vi "UHR-Fleezers Control (host) - 12.2.vi"() -> ()   [LabVIEW 2014] (continued)
            n2614 = xnode "Read/Write Control"("FPGA VI Reference In"=w4956, "error in"=w4955, "AI to FIFO"=w4959, "APD to FIFO"=w4959, "Start scan"=w4959, "Start scan (MCL)"=w4959) -> ("FPGA VI Reference Out"=w4961:T22, "error out"=w4960:errorcluster)
          }
        }
        "Raster Scanning..." <- TRUE ("Scanning...")
      }
    }
    n2615 = local read "Flushing P3"() -> (w3736:bool)
    n2616 = case "Keep track of when Harvard Pump 3 is done flushing" shown="True" w3736 {
      frame False {
      }
      frame True {
        n2617 = local read "Flush rate (uL/m) P3"() -> (w4119:dbl)
        n2618 = local read "DMA Update Period (s)"() -> (w4113:dbl)
        n2619 = local read "HP3 Flush Time (s)"() -> (w4127:dbl)
        n2620 = Divide(x=w4119, y=60.0) -> (x/y=w4114:dbl)
        n2621 = feedback #6(0) -> (w4125:i32)
        n2622 = Increment(x=w4125) -> (x+1=w4120:i32)
        n2623 = Divide(x=w4127, y=w4113) -> (x/y=w4121:dbl)
        n2624 = Multiply(x=w4113, y=w4114) -> (x*y=w4112:dbl)
        n2625 = Greater?(x=w4120, y=w4121) -> (0:w4124:bool)
        n2626 = feedback #7(0.0) -> (w4115:dbl)
        n2627 = Compound Arithmetic op=MULTIPLY(w4113, w4120, w4114) -> (→"P3 Flush Volume (uL)":dbl)
        n2628 = case shown="True" w4124 {
          tunnel: w4120 -> [w4128 _]
          tunnel: [w4128 0] -> w4123
          frame False {
          }
          frame True {
            w4129 = FALSE ("Flushing P3")
            n2629 = local write "Inject Pump 3"(w4129) -> ()
            n2630 = local write "Flushing P3"(w4129) -> ()
            n2631 = property on="Clear Volume P3" class="Bool (strict)"("Val(Sgnl)"=TRUE ("Value (Signaling)")) -> ()  [unwired: 2 in, 2 out]
          }
        }
        n2632 = feedback-in #6(w4123) -> ()
        n2633 = Divide(x=w4120, y=w4121) -> (x/y=→"P3 Flushing Bar":dbl)
        n2634 = Add(x=w4112, y=w4115) -> (x+y=w4116:dbl)
        "Total Volume\nFlowed P3 (uL)" <- w4116
        n2635 = feedback-in #7(w4116) -> ()
      }
    }
    n2636 = And(x="Save scans", y=w3954) -> (x .and. y?=w3993:bool)
    n2637 = local read "Flushing samp"() -> (w3729:bool)
    n2638 = case shown="True" w3729 {
      frame False {
      }
      frame True {
        n2639 = local read "DMA Update Period (s)"() -> (w4072:dbl)
        n2640 = local read "Flush rate (mL/m)"() -> (w4084:dbl)
        n2641 = local read "Samp Flush Time (s)"() -> (w4085:dbl)
        n2642 = Divide(x=w4084, y=60.0) -> (x/y=w4071:dbl)
        n2643 = feedback #8(0) -> (w4077:i32)
        n2644 = Increment(x=w4077) -> (x+1=w4076:i32)
        n2645 = Divide(x=w4085, y=w4072) -> (x/y=w4081:dbl)
        n2646 = Multiply(x=w4072, y=w4071) -> (x*y=w4070:dbl)
        n2647 = Greater?(x=w4076, y=w4081) -> (0:w4080:bool)
        n2648 = feedback #9(0.0) -> (w4073:dbl)
        n2649 = Compound Arithmetic op=MULTIPLY(w4072, w4076, w4071) -> (→"Samp Volume (uL)":dbl)
        n2650 = Divide(x=w4076, y=w4081) -> (x/y=→"Samp flush bar":dbl)
        n2651 = case shown="True" w4080 {
          tunnel: [w4086 0] -> w4079
          tunnel: w4076 -> [w4086 _]
          frame False {
          }
          frame True {
            w4089 = FALSE ("Flushing samp")
            n2652 = local write "Sample Channel\nFlow"(w4089) -> ()
            n2653 = local write "Flushing samp"(w4089) -> ()
            n2654 = property on="Clear Volume" class="Bool (strict)"("Val(Sgnl)"=TRUE) -> ()  [unwired: 2 in, 2 out]
          }
        }
        n2655 = feedback-in #8(w4079) -> ()
        n2656 = Add(x=w4070, y=w4073) -> (x+y=w4074:dbl)
        "Total Volume\nFlowed Samp (uL)" <- w4074
        n2657 = feedback-in #9(w4074) -> ()
      }
    }
    n2658 = Compound Arithmetic op=OR("Start MCL Scan", "Confocal\nImage", "Confocal\nLinescan") -> (w3952:bool)
    n2659 = And(x="Save Data (MCL)", y=w3952) -> (x .and. y?=w3992:bool)
    n2660 = case "Start MCL raster scan" shown="True" w3952 {
      tunnel: w3720 -> [w4534 w4550]
      tunnel: w3994 -> [w4533 w4549]
      tunnel: [w4534 w4545] -> w3727
      tunnel: [w4533 w4544] -> w3725
      tunnel: [FALSE w4543] -> w3978
      tunnel: "Start MCL Scan" -> [_ w4538]
      tunnel: "Confocal\nImage" -> [_ w4537]
      tunnel: "Confocal\nLinescan" -> [_ _]
      frame False {
      }
      frame True {
        w4543 = TRUE
        n2661 = case shown="True" "Restart DMA? (MCL)" {
          tunnel: [w4595 w4597] -> w4548
          tunnel: [w4594 w4596] -> w4547
          tunnel: w4550 -> [w4595 w4600]
          tunnel: w4549 -> [w4594 w4599]
          frame False {
          }
          frame True {
            n2662 = call "reset FPGA DMA.vi"("error in"=w4599, "FPGA VI Reference In"=w4600) -> ("error out"=w4596:errorcluster, "FPGA VI Reference Out"=w4597:T22)
            n2663 = local write "Overflow (data lost)"(FALSE ("Overflow (data lost)")) -> ()
          }
        }
        n2664 = case shown="False" w4538 {
          selector: w4538 -> [_ w4554]
          tunnel: w4537 -> [w4553 _]
          tunnel: [w4553 w4554] -> w4536
          frame False {
            n2665 = property on="2D or 1D Scan" class="Bool (strict)"("Val(Sgnl)"=w4553) -> ()  [unwired: 2 in, 2 out]
            n2666 = property on="Confocal\nImage" class="Bool (strict)"("Value"=FALSE ("Start Confocal Map")) -> ()  [unwired: 2 in, 2 out]
          }
          frame True {
          }
        }
        n2667 = local write "MCL Scanning"(w4543) -> ()
        n2668 = local read "AO1"() -> (w4540:dbl)
        n2669 = local read "AO2"() -> (w4539:dbl)
        n2670 = case shown="True" "Center Scan" {
          tunnel: w4548 -> [w4561 w4593]
          tunnel: w4547 -> [w4560 w4592]
          tunnel: [w4559 w4591] -> w4545
          tunnel: [w4558 w4590] -> w4544
          tunnel: [w4556 w4577] -> w4542
          tunnel: [w4555 w4576] -> w4541
          tunnel: w4540 -> [w4556 w4582]
          tunnel: w4539 -> [w4555 w4585]
          tunnel: w4536 -> [_ _]
          frame False {
            w4557 = TRUE ("AI to FIFO")
            n2671 = xnode "Read/Write Control"("FPGA VI Reference In"=w4561, "error in"=w4560, "AI to FIFO"=w4557, "APD to FIFO"=w4557, "Start scan (MCL)"=w4557) -> ("FPGA VI Reference Out"=w4559:T22, "error out"=w4558:errorcluster)
          }
          frame True {
            w4589 = TRUE ("AI to FIFO")
            n2672 = local read "Scan steps (MCL)"() -> (w4568:u64)
            n2673 = local read "Scan lines (y)"() -> (w4564:u64)
            n2674 = local read "Fast Scan Dir"() -> (w4575:bool)
            n2675 = local read "Actual MCL Inc (V)"() -> (w4565:dbl)
            n2676 = Decrement(x=w4564) -> (x-1=w4563:u64)
            n2677 = Decrement(x=w4568) -> (x-1=w4567:u64)
            n2678 = Multiply(x=w4565, y=w4563) -> (x*y=w4562:dbl)
            n2679 = Divide(x=w4562, y=2.0) -> (x/y=w4572:dbl)
            n2680 = Multiply(x=w4565, y=w4567) -> (x*y=w4566:dbl)
            n2681 = Divide(x=w4566, y=2.0) -> (x/y=w4571:dbl)
            n2682 = Select(t=w4571, s=w4575, f=w4572) -> (s? t:f=w4570:dbl)
            n2683 = Select(t=w4572, s=w4575, f=w4571) -> (s? t:f=w4574:dbl)
            n2684 = Subtract(x=w4582, y=w4574) -> (x-y=w4573:dbl)
            n2685 = Subtract(x=w4585, y=w4570) -> (x-y=w4569:dbl)
            n2686 = local read "2D or 1D Scan"() -> (w4587:bool)
            n2687 = Not(x=w4575) -> (.not. x?=w4581:bool)
            n2688 = Not(x=w4587) -> (.not. x?=w4583:bool)
            n2689 = And(x=w4575, y=w4583) -> (x .and. y?=w4584:bool)
            n2690 = And(x=w4583, y=w4581) -> (x .and. y?=w4586:bool)
            n2691 = Select(t=w4585, s=w4586, f=w4569) -> (s? t:f=w4576:dbl)
            n2692 = Select(t=w4582, s=w4584, f=w4573) -> (s? t:f=w4577:dbl)
            n2693 = call "Volt to I16.vi"("Voltage In"=w4577) -> ("I16 Voltage Out"=w4580:i16)
            n2694 = call "Volt to I16.vi"("Voltage In"=w4576) -> ("I16 Voltage Out"=w4579:i16)
            n2695 = xnode "Read/Write Control"("FPGA VI Reference In"=w4593, "error in"=w4592, "AI to FIFO"=w4589, "APD to FIFO"=w4589, "Start scan (MCL)"=w4589, "AO1"=w4580, "AO2"=w4579) -> ("FPGA VI Reference Out"=w4591:T22, "error out"=w4590:errorcluster)
          }
        }
        "Initial Y" <- w4542
        "Initial X" <- w4541
        n2696 = local write "Tab Control 6"(T3."Imaging" ("Tab Control 6")) -> ()
        "wait to reset values" <- w4543
      }
    }
    n2697 = case shown="True" "Wiggle" {
      selector: "Wiggle" -> [w4043 _]
      tunnel: w3727 -> [w4045 w4058]
      tunnel: [w4042 w4061] -> w3726
      tunnel: w3725 -> [w4044 w4056]
      tunnel: [w4041 w4060] -> w3724
      frame False {
        n2698 = xnode "Read/Write Control"("FPGA VI Reference In"=w4045, "error in"=w4044, "Wiggle trap 1"=w4043) -> ("FPGA VI Reference Out"=w4042:T22, "error out"=w4041:errorcluster)
      }
      frame True {
        w4050 = FALSE ("Abort wiggle")
        w4054 = TRUE
        n2699 = local read "Restart DMA? (AOD)"() -> (w4059:bool)
        n2700 = case shown="True" w4059 {
          tunnel: w4058 -> [w4063 w4068]
          tunnel: [w4063 w4067] -> w4057
          tunnel: w4056 -> [w4062 w4066]
          tunnel: [w4062 w4065] -> w4055
          frame False {
          }
          frame True {
            n2701 = local write "Overflow (data lost)"(FALSE) -> ()
            n2702 = call "reset FPGA DMA.vi"("error in"=w4066, "FPGA VI Reference In"=w4068) -> ("error out"=w4065:errorcluster, "FPGA VI Reference Out"=w4067:T22)
          }
        }
        n2703 = local write "Wiggle"(FALSE) -> ()
        n2704 = xnode "Read/Write Control"("FPGA VI Reference In"=w4057, "error in"=w4055, "AI to FIFO"=w4054, "APD to FIFO"=w4054, "Wiggle trap 1"="Wiggle T1", "Wiggle freq 1 (Hz)"="Wiggle freq 1 (Hz)", "Wiggle amp 1"="Wiggle amp 1 (units?)", "Abort wiggle 1"=w4050, "Wiggle trap 2"="Wiggle T2", "Abort wiggle 2"=w4050, "Wiggle freq 2 (Hz)"="Wig Freq 2 (Hz)", "Wiggle amp 2"="Wig amp 2") -> ("FPGA VI Reference Out"=w4061:T22, "error out"=w4060:errorcluster)
      }
    }
    n2705 = local read "Trap Pos Elements/DMA read"() -> (w3710:u32)
    n2706 = local read "Trap AI Elements/DMA read"() -> (w3704:u32)
    n2707 = local read "APD Elements/DMA read"() -> (w3712:u32)
    n2708 = xnode "Get APD Data"("FPGA VI Reference In"=w3726, "error in"=w3724, "Number of Elements"=w3712, "Timeout (ms)"=-1) -> ("Data"=w3888:u32[], "Elements Remaining"=→"APD FIFO Elements Remaining":u32)  [unwired: 2 out]
    n2709 = xnode "Invoke Method"("FPGA VI Reference In"=w3726, "error in"=w3724, "Number of Elements"=w3710, "Timeout (ms)"=-1) -> ("Data"=w3819:u16[], "Elements Remaining"=→"Trap Pos FIFO El Remaining":u32)  [unwired: 2 out]
    n2710 = xnode "Get Trap Data"("FPGA VI Reference In"=w3726, "error in"=w3724, "Number of Elements"=w3704, "Timeout (ms)"=-1 ("Timeout")) -> ("FPGA VI Reference Out"=w3757:T22, "error out"=w3756:errorcluster, "Data"=w3820:i16[], "Elements Remaining"=w3703:u32)
    "FIFO El. Rem." <- w3703
    n2711 = local read "Trap AI FIFO Depth"() -> (w4038:u32)
    n2712 = Subtract(x=w4038, y=w3704) -> (x-y=w4037:u32)
    n2713 = Decimate 1D Array(w3819) -> (w3708:u16[], w3706:u16[], w3707:u16[])
    n2714 = Divide(x=w3703, y=w4037) -> (x/y=w4036:dbl)
    "Buffer Status" <- w4036
    n2715 = To Unsigned Long Integer(number=w3708) -> (unsigned 32bit integer=w3818:u32[])
    n2716 = Join Numbers(hi=w3706, lo=w3707) -> ((hi.lo)=w3817:u32[])
    n2717 = Equal?(x=w4036, y=1.0) -> (x = y?=w4034:bool)
    n2718 = Join Numbers(hi=w3818, lo=w3817) -> ((hi.lo)=w3811:u64[])
    n2719 = call "IR AOM word to freq - vec.vi"("Frequency Word In (double vec)"=w3811) -> ("Frequency Out"=w3854:dbl[])
    n2720 = case "Alert buffer overflow" shown="True" w4034 {
      frame False {
      }
      frame True {
        n2721 = call <vilib>:"Beep.vi"() -> ()  [unwired: 3 in, 9 out]
        "Overflow (data lost)" <- TRUE ("Overflow (data lost)")
      }
    }
    n2722 = Decimate 1D Array(w3854) -> (w3853:dbl[], w3852:dbl[])
    n2723 = Build Array(w3853, w3852) -> (w3851:dbl[][])
    n2724 = local read "Trap Sets"() -> (w3918:u32)
    n2725 = case "Deinterlace trap data, average down PSD" shown="2" w3918 {
      tunnel: w3820 -> [w4626 w4695]
      tunnel: [w4629 w4692] -> w3911
      tunnel: [w4626 w4694] -> w3814
      tunnel: "Detector Type" -> [w4631 w4690]
      tunnel: [w4630 w4693] -> w3910
      tunnel: [w4628 w4691] -> w4011
      frame 1, Default {
        n2726 = Divide(x=w4626, y=3276.7) -> (x/y=w4627:dbl[])
        n2727 = Decimate 1D Array(w4627) -> (w4640:dbl[], w4639:dbl[], w4638:dbl[], w4637:dbl[], w4636:dbl[], w4635:dbl[], w4634:dbl[], w4633:dbl[])
        n2728 = case shown="\"IR-QPD + PSD + FB-QPD position\"" w4631 {
          tunnel: w4640 -> [w4664 w4689]
          tunnel: w4639 -> [w4663 w4688]
          tunnel: w4638 -> [w4648 w4666]
          tunnel: w4637 -> [w4649 w4676]
          tunnel: w4636 -> [w4662 w4687]
          tunnel: w4635 -> [w4661 w4686]
          tunnel: w4634 -> [w4645 w4667]
          tunnel: w4633 -> [w4644 w4665]
          tunnel: [w4643 w4673] -> w4630
          tunnel: [w4642 w4672] -> w4629
          tunnel: [w4641 w4671] -> w4628
          frame "IR-QPD + PSD + FB-QPD", Default {
            w4641 = 0  # Channel pattern
            n2729 = Divide(x=w4664, y=w4649) -> (x/y=w4651:dbl[])
            n2730 = Divide(x=w4663, y=w4649) -> (x/y=w4650:dbl[])
            n2731 = Divide(x=w4662, y=w4645) -> (x/y=w4647:dbl[])
            n2732 = Divide(x=w4661, y=w4644) -> (x/y=w4646:dbl[])
            n2733 = Build Array(w4651, w4650, w4649, w4648, w4647, w4646, w4645, w4644) -> (w4642:dbl[][])
            n2734 = Bundle("T1 Y", "T1 X", "T1 Sum", "FB Sum", "PSD Y", "PSD X", "PSD Y Sum", "PSD X Sum") -> (w4660:T47)  [unwired: 1 out]
            n2735 = Cluster To Array(cluster=w4660) -> (array=w4643:string[])
          }
          frame "IR-QPD + PSD + FB-QPD position" {
            w4671 = 3  # Channel pattern
            n2736 = Negate(x=w4667) -> (-x=w4668:dbl[])
            n2737 = Divide(x=w4689, y=w4676) -> (x/y=w4678:dbl[])
            n2738 = Divide(x=w4688, y=w4676) -> (x/y=w4677:dbl[])
            n2739 = Divide(x=w4687, y=w4667) -> (x/y=w4675:dbl[])
            n2740 = Divide(x=w4686, y=w4668) -> (x/y=w4674:dbl[])
            n2741 = Build Array(w4678, w4677, w4676, w4665, w4666, w4675, w4674, w4667) -> (w4672:dbl[][])
            n2742 = Bundle("T1 Y", "T1 X", "T1 Sum", "FB X", "FB Sum", "PSD Y", "PSD X", "PSD Y Sum") -> (w4685:T47)  [unwired: 1 out]
            n2743 = Cluster To Array(cluster=w4685) -> (array=w4673:string[])
          }
        }
      }
      frame 2 {
        n2744 = case shown="\"IR-QPD + PSD + FB-QPD XY positions\"" w4690 {
          tunnel: w4695 -> [w4757 w4824 w4893]
          tunnel: [w4708 w4820 w4838] -> w4694
          tunnel: [w4733 w4812 w4879] -> w4693
          tunnel: [w4732 w4779 w4850] -> w4692
          tunnel: [w4728 w4810 w4877] -> w4691
          frame "IR-QPD + PSD + FB-QPD", Default {
            w4728 = 1  # Channel pattern
            # "time average x2 the 4th signal and the 4 psd signals (detection laser)"
            # "deinterlace 3 signals from qpd"
            n2745 = Decimate 1D Array(w4757) -> (w4756:i16[], w4755:i16[], w4731:i16[], w4754:i16[], w4707:i16[], w4706:i16[], w4705:i16[], w4704:i16[])
            n2746 = Decimate 1D Array(w4731) -> (w4697:i16[], w4696:i16[])
            n2747 = Decimate 1D Array(w4756) -> (w4703:i16[], w4702:i16[])
            n2748 = Decimate 1D Array(w4755) -> (w4701:i16[], w4699:i16[])
            n2749 = Decimate 1D Array(w4754) -> (w4700:i16[], w4698:i16[])
            n2750 = call "downsample 1D array - double.vi"("Ave N"=2.0, "Array In"=w4707) -> ("Array Out"=w4749:dbl[])  [unwired: 1 out]
            n2751 = call "downsample 1D array - double.vi"("Ave N"=2.0, "Array In"=w4706) -> ("Array Out"=w4734:dbl[])  [unwired: 1 out]
            n2752 = call "downsample 1D array - double.vi"("Ave N"=2.0, "Array In"=w4705) -> ("Array Out"=w4748:dbl[])  [unwired: 1 out]
            n2753 = call "downsample 1D array - double.vi"("Ave N"=2.0, "Array In"=w4704) -> ("Array Out"=w4747:dbl[])  [unwired: 1 out]
            n2754 = Interleave 1D Arrays(w4703, w4701, w4700, w4702, w4699, w4698, w4697, w4696, w4749, w4734, w4748, w4747) -> (w4746:dbl[])
            n2755 = Divide(x=w4746, y=3276.7) -> (x/y=w4745:dbl[])
            n2756 = Decimate 1D Array(w4745) -> (w4744:dbl[], w4743:dbl[], w4742:dbl[], w4741:dbl[], w4740:dbl[], w4739:dbl[], w4730:dbl[], w4729:dbl[], w4738:dbl[], w4737:dbl[], w4736:dbl[], w4735:dbl[])
            n2757 = Divide(x=w4744, y=w4742) -> (x/y=w4715:dbl[])
            n2758 = Divide(x=w4743, y=w4742) -> (x/y=w4714:dbl[])
            n2759 = Divide(x=w4741, y=w4739) -> (x/y=w4713:dbl[])
            n2760 = Divide(x=w4740, y=w4739) -> (x/y=w4712:dbl[])
            n2761 = Divide(x=w4738, y=w4736) -> (x/y=w4711:dbl[])
            n2762 = Divide(x=w4737, y=w4735) -> (x/y=w4710:dbl[])
            n2763 = Build Array(w4715, w4714, w4742, w4713, w4712, w4739, w4730, w4729, w4711, w4710, w4736, w4735) -> (w4732:dbl[][])
            n2764 = Bundle("T1 Y", "T1 X", "T1 Sum", "T2 Y", "T2 X", "T2 Sum", "T1 FB Sum", "T2 FB Sum", "PSD Y", "PSD X", "PSD Y Sum", "PSD X Sum") -> (w4716:T48)  [unwired: 1 out]
            n2765 = To Word Integer(number=w4746) -> (16bit integer=w4708:i16[])
            n2766 = Cluster To Array(cluster=w4716) -> (array=w4733:string[])
          }
          frame "IR-QPD + PSD + FB-QPD X position" {
            w4810 = 2  # Channel pattern
            # "time average x2 the 3 psd signals (detection laser)"
            # "deinterlace 3 signals from qpds"
            n2767 = Decimate 1D Array(w4824) -> (w4823:i16[], w4822:i16[], w4811:i16[], w4821:i16[], w4771:i16[], w4770:i16[], w4769:i16[], w4798:i16[])
            n2768 = Decimate 1D Array(w4811) -> (w4761:i16[], w4759:i16[])
            n2769 = Decimate 1D Array(w4823) -> (w4768:i16[], w4765:i16[])
            n2770 = Decimate 1D Array(w4822) -> (w4767:i16[], w4764:i16[])
            n2771 = Decimate 1D Array(w4821) -> (w4766:i16[], w4763:i16[])
            n2772 = Decimate 1D Array(w4798) -> (w4762:i16[], w4760:i16[])
            n2773 = call "downsample 1D array - I16.vi"("Ave N"=2.0, "Array In"=w4771) -> ("Array Out"=w4776:i16[])  [unwired: 1 in]
            n2774 = call "downsample 1D array - I16.vi"("Ave N"=2.0, "Array In"=w4769) -> ("Array Out"=w4772:i16[])  [unwired: 1 in]
            n2775 = call "downsample 1D array - I16.vi"("Ave N"=2.0, "Array In"=w4770) -> ("Array Out"=w4774:i16[])  [unwired: 1 in]
            n2776 = Interleave 1D Arrays(w4768, w4767, w4766, w4765, w4764, w4763, w4762, w4761, w4760, w4759, w4776, w4774, w4772) -> (w4820:i16[])
            n2777 = Divide(x=w4820, y=3276.7) -> (x/y=w4819:dbl[])
            n2778 = Decimate 1D Array(w4819) -> (w4818:dbl[], w4817:dbl[], w4816:dbl[], w4815:dbl[], w4814:dbl[], w4813:dbl[], w4790:dbl[], w4788:dbl[], w4787:dbl[], w4785:dbl[], w4784:dbl[], w4783:dbl[], w4780:dbl[])
            n2779 = Negate(x=w4780) -> (-x=w4778:dbl[])
            n2780 = Divide(x=w4784, y=w4780) -> (x/y=w4782:dbl[])
            n2781 = Divide(x=w4783, y=w4778) -> (x/y=w4781:dbl[])
            n2782 = Divide(x=w4818, y=w4816) -> (x/y=w4802:dbl[])
            n2783 = Divide(x=w4817, y=w4816) -> (x/y=w4801:dbl[])
            n2784 = Divide(x=w4815, y=w4813) -> (x/y=w4800:dbl[])
            n2785 = Divide(x=w4814, y=w4813) -> (x/y=w4799:dbl[])
            n2786 = Divide(x=w4790, y=w4788) -> (x/y=w4789:dbl[])
            n2787 = Divide(x=w4787, y=w4785) -> (x/y=w4786:dbl[])
            n2788 = Build Array(w4802, w4801, w4816, w4800, w4799, w4813, w4789, w4788, w4786, w4785, w4782, w4781, w4780) -> (w4779:dbl[][])
            n2789 = Bundle("T1 Y", "T1 X", "T1 Sum", "T2 Y", "T2 X", "T2 Sum", "T1 FB X", "T1 FB Sum", "T2 FB X", "T2 FB Sum", "PSD Y", "PSD X", "PSD Y Sum") -> (w4803:T49)  [unwired: 1 out]
            n2790 = Cluster To Array(cluster=w4803) -> (array=w4812:string[])
          }
          frame "IR-QPD + PSD + FB-QPD XY positions" {
            w4877 = 4  # Channel pattern
            # "time average x2 the 3 psd signals (detection laser)"
            # "deinterlace 3 signals from qpds"
            n2791 = Decimate 1D Array(w4893) -> (w4892:i16[], w4891:i16[], w4878:i16[], w4890:i16[], w4848:i16[], w4866:i16[])  [unwired: 2 out]
            n2792 = Decimate 1D Array "Feedback Sum"(w4878) -> (w4829:i16[], w4826:i16[])
            n2793 = Decimate 1D Array "QPD Y"(w4892) -> (w4837:i16[], w4834:i16[])
            n2794 = Decimate 1D Array "QPD X"(w4891) -> (w4836:i16[], w4833:i16[])
            n2795 = Decimate 1D Array "Feedback Y"(w4848) -> (w4831:i16[], w4828:i16[])
            n2796 = Decimate 1D Array "QPD Sum"(w4890) -> (w4835:i16[], w4832:i16[])
            n2797 = Decimate 1D Array "Feedback X"(w4866) -> (w4830:i16[], w4827:i16[])
            n2798 = call "downsample 1D array - double.vi"("Ave N"=2.0) -> ("Array Out"=w4865:dbl[])  [unwired: 1 in, 1 out]
            n2799 = call "downsample 1D array - double.vi"("Ave N"=2.0) -> ("Array Out"=w4864:dbl[])  [unwired: 1 in, 1 out]
            n2800 = Interleave 1D Arrays(w4837, w4836, w4835, w4834, w4833, w4832, w4831, w4830, w4829, w4828, w4827, w4826, w4865, w4864) -> (w4887:dbl[])
            n2801 = Divide(x=w4887, y=3276.7) -> (x/y=w4886:dbl[])
            n2802 = Decimate 1D Array(w4886) -> (w4885:dbl[], w4884:dbl[], w4883:dbl[], w4882:dbl[], w4881:dbl[], w4880:dbl[], w4845:dbl[], w4857:dbl[], w4843:dbl[], w4844:dbl[], w4855:dbl[], w4841:dbl[], w4853:dbl[], w4851:dbl[])
            n2803 = Negate(x=w4851) -> (-x=w4849:dbl[])
            n2804 = Divide(x=w4853, y=w4849) -> (x/y=w4852:dbl[])
            n2805 = Divide(x=w4844, y=w4841) -> (x/y=w4840:dbl[])
            n2806 = Divide(x=w4845, y=w4843) -> (x/y=w4842:dbl[])
            n2807 = Divide(x=w4885, y=w4883) -> (x/y=w4870:dbl[])
            n2808 = Divide(x=w4884, y=w4883) -> (x/y=w4869:dbl[])
            n2809 = Divide(x=w4882, y=w4880) -> (x/y=w4868:dbl[])
            n2810 = Divide(x=w4881, y=w4880) -> (x/y=w4867:dbl[])
            n2811 = Divide(x=w4857, y=w4843) -> (x/y=w4856:dbl[])
            n2812 = Divide(x=w4855, y=w4841) -> (x/y=w4854:dbl[])
            n2813 = Build Array(w4870, w4869, w4883, w4868, w4867, w4880, w4842, w4856, w4843, w4840, w4854, w4841, w4852, w4851) -> (w4850:dbl[][])
            n2814 = Bundle("T1 Y", "T1 X", "T1 Sum", "T2 Y", "T2 X", "T2 Sum", "T1 FB Y", "T1 FB X", "T1 FB Sum", "T2 FB Y", "T2 FB X", "T2 FB Sum", "PSD X", "PSD Y Sum") -> (w4839:T50)  [unwired: 1 out]
            n2815 = To Word Integer(number=w4887) -> (16bit integer=w4838:i16[])
            n2816 = Cluster To Array(cluster=w4839) -> (array=w4879:string[])
          }
        }
      }
    }
    "AI labels" <- w3910
    n2817 = Decimate 1D Array(w3888) -> (w3698:u32[], w3699:u32[])
    n2818 = local read "DMA Update Period (s)"() -> (w3919:dbl)
    n2819 = Build Array(w3698, w3699) -> (w3702:u32[][])
    n2820 = local read "Data Period (s)"() -> (w3773:dbl)
    n2821 = local read "BD 1 Frequency 2 (MHz)"() -> (w3806:dbl)
    n2822 = local read "BD 1 Frequency 1 (MHz)"() -> (w3807:dbl)
    n2823 = Decimate 1D Array(w3814) -> (w3834:i16[], w3833:i16[], w3831:i16[], w3830:i16[])  [unwired: 9 out]
    n2824 = To Double Precision Float(number=w3702) -> (double precision float=w3976:dbl[][])
    n2825 = local read "APD Integration Time (s)"() -> (w3870:dbl)
    n2826 = Multiply(x=w3773, y="Trap Pos. Disp. Downsample") -> (x*y=w3771:dbl)
    n2827 = Divide(x=w3834, y=w3833) -> (x/y=w3835:dbl[])
    n2828 = Divide(x=w3831, y=w3830) -> (x/y=w3832:dbl[])
    n2829 = feedback #10(0.0) -> (w3848:dbl)
    n2830 = Add(x=w3919, y=w3848) -> (x+y=w4013:dbl)
    n2831 = feedback-in #10(w4013) -> ()
    n2832 = local read "AOM X Cal (nm/MHz)"() -> (w3804:dbl)
    n2833 = To Time Stamp(1:w3848) -> (0:w3847:timestamp)
    n2834 = Split 1D Array(array=w3835, index="N El. to Ave.") -> (second subarray=w3838:dbl[])  [unwired: 1 out]
    n2835 = Split 1D Array(array=w3832, index="N El. to Ave.") -> (second subarray=w3837:dbl[])  [unwired: 1 out]
    n2836 = Multiply(x=w3773, y="Trap Disp. Downsample") -> (x*y=w3849:dbl)
    "Display Period (s)" <- w3849
    n2837 = for "Trap AI" {
      tunnel: [w4625] -> w4007 mode=indexing
      tunnel: w3847 -> [w4615]
      tunnel: "Trap Disp. Downsample" -> [w4623]
      tunnel: w3911 -> [w4621] mode=indexing
      tunnel: w3773 -> [w4620]
      tunnel: w3910 -> [w4619] mode=indexing
      tunnel: w3846 -> [w4618]
      tunnel: [w4617] -> w3880 mode=indexing
      tunnel: w3849 -> [w4616]
      workers-P: _ -> [_]
      n2838 = Bundle By Name("Y"=w4621, "dt"=w4620) -> (w4622:waveform(dbl))  [unwired: 1 out]
      n2839 = Set Waveform Attribute(5:w4619, 6:w4618, 7:w4622) -> (3:w4617:waveform(dbl))  [unwired: 1 in, 2 out]
      n2840 = call "downsample 1D array - double.vi"("Ave N"=w4623, "Array In"=w4621) -> ("Array Out"=w4624:dbl[])  [unwired: 1 out]
      n2841 = Bundle By Name(cluster=w4617, "t0"=w4615, "Y"=w4624, "dt"=w4616) -> (w4625:waveform(dbl))
    }
    n2842 = Bundle("BD 1 Frequency 1 (MHz)"=w3807, "BD 1 Frequency 2 (MHz)"=w3806) -> (w3808:T51)  [unwired: 1 out]
    n2843 = call-poly <vilib>:"Mean.vi"("X"=w3837) -> ("mean"=w3825:dbl)  [unwired: 1 out]
    n2844 = call-poly <vilib>:"Mean.vi"("X"=w3838) -> ("mean"=w3826:dbl)  [unwired: 1 out]
    n2845 = Reciprocal(x=w3849) -> (1/x=→"Trap Disp. Freq. (Hz)":dbl)
    n2846 = Cluster To Array(cluster=w3808) -> (array=w3805:dbl[])
    n2847 = local read "Trap X AI1 (DMA)"() -> (w3836:T13)
    n2848 = local read "Data points/scans (MCL)"() -> (w3987:dbl)
    n2849 = To Fixed-Point(number=w3825) -> (fixed-point=w3823:fxp<+/-,16,1>)  [unwired: 1 in]
    n2850 = To Fixed-Point(number=w3826) -> (fixed-point=w3824:fxp<+/-,16,1>)  [unwired: 1 in]
    n2851 = Bundle("Trap 1 Pos.", "Trap 2 Pos.") -> (w3845:cluster{string, string})  [unwired: 1 out]
    n2852 = Bundle By Name(cluster=w3836, "Set 1"=w3824, "Set 2"=w3823) -> (→"Trap X AI1 (DMA)":T13)
    n2853 = Cluster To Array(cluster=w3845) -> (array=w3842:string[])
    n2854 = Bundle("APD 1", "APD 2") -> (w4006:cluster{string, string})  [unwired: 1 out]
    n2855 = Select(t=-1.0, s="Negate Y Axis", f=1.0) -> (s? t:f=w3790:dbl)
    n2856 = for "Trap Position" {
      tunnel: w3851 -> [w4257] mode=indexing
      tunnel: "Trap Pos. Disp. Downsample" -> [w4256]
      tunnel: w3771 -> [w4254]
      tunnel: w3847 -> [w4253]
      tunnel: w3846 -> [w4251]
      tunnel: w3842 -> [w4250] mode=indexing
      tunnel: [w4249] -> w3760 mode=indexing
      tunnel: w3805 -> [w4247] mode=indexing
      tunnel: w3804 -> [w4245]
      tunnel: w3790 -> [w4244]
      n2857 = call "downsample 1D array - double.vi"("Ave N"=w4256, "Array In"=w4257) -> ("Array Out"=w4255:dbl[])  [unwired: 1 out]
      n2858 = Subtract(x=w4255, y=w4247) -> (x-y=w4248:dbl[])
      n2859 = Multiply(x=w4245, y=w4248) -> (x*y=w4246:dbl[])
      n2860 = Multiply(x=w4244, y=w4246) -> (x*y=w4243:dbl[])
      n2861 = Bundle By Name("Y"=w4243, "dt"=w4254, "t0"=w4253) -> (w4252:waveform(dbl))  [unwired: 1 out]
      n2862 = Set Waveform Attribute(5:w4250, 6:w4251, 7:w4252) -> (3:w4249:waveform(dbl))  [unwired: 1 in, 2 out]
    }
    n2863 = Cluster To Array(cluster=w4006) -> (array=w4003:string[])
    n2864 = for "APD" {
      tunnel: w3976 -> [w4601] mode=indexing
      tunnel: w3870 -> [w4612]
      tunnel: [w4608] -> w3876 mode=indexing
      tunnel: "APD Disp. Scale" -> [w4609]
      tunnel: w3846 -> [w4607]
      tunnel: w4003 -> [w4606] mode=indexing
      tunnel: "APD Disp. Downsample" -> [w4603]
      tunnel: [w4605] -> w4002
      workers-P: _ -> [_]
      tunnel: w3847 -> [w4602]
      n2865 = call "integrate 1D array interval - double.vi"("Ave N"=w4603, "Array In"=w4601) -> ("Array Out"=w4604:dbl[])  [unwired: 1 out]
      n2866 = Multiply(x=w4612, y=w4603) -> (x*y=w4605:dbl)
      n2867 = Divide(x=w4604, y=w4609) -> (x/y=w4610:dbl[])
      n2868 = Bundle By Name("t0"=w4602, "Y"=w4610, "dt"=w4605) -> (w4611:waveform(dbl))  [unwired: 1 out]
      n2869 = Set Waveform Attribute(5:w4606, 6:w4607, 7:w4611) -> (3:w4608:waveform(dbl))  [unwired: 1 in, 2 out]
    }
    "APD Display Period (s)" <- w4002
    n2870 = Reciprocal(x=w4002) -> (1/x=→"APD Display Freq. (Hz)":dbl)
    n2871 = local read "Display Period (s)"() -> (w3897:dbl)
    n2872 = Increment(x=w3987) -> (x+1=w3988:dbl)
    n2873 = To Double Precision Float(number=w3698) -> (double precision float=w3908:dbl[])
    n2874 = Index Array(array=w3760, index=0) -> (element=w3764:waveform(dbl))
    n2875 = Index Array(array=w3760, index=1) -> (element=w3759:waveform(dbl))
    n2876 = feedback #11(w3988) -> (w3991:dbl)
    n2877 = Select(t=0, s=w3978, f=w3991) -> (s? t:f=w3984:dbl)
    n2878 = Array Size(array=w3908) -> (size(s)=w3990:i32)
    n2879 = Add(x=w3990, y=w3984) -> (x+y=w3985:dbl)
    n2880 = Unbundle By Name(w3764) -> ("Y"=w3765:dbl[])
    n2881 = feedback #12(w3698) -> (w3975:u32[])
    n2882 = Build Array (concatenate)(w3975, w3698) -> (w3972:u32[])
    n2883 = feedback #13(w3699) -> (w3875:u32[])
    n2884 = Divide(x="Bead Sep. Int. Time (s)", y=w3897) -> (x/y=w3800:dbl)
    n2885 = Build Array (concatenate)(w3875, w3699) -> (w3874:u32[])
    n2886 = Add(x=w3765, y="FB Trap Pos Offset") -> (x+y=w3763:dbl[])
    "T1 x pos data" <- w3763
    n2887 = Greater?(x=w3985, y=w3987) -> (0:w3986:bool)
    n2888 = feedback #14(w3763) -> (w3802:dbl[])
    n2889 = Build Array (concatenate)(w3763, w3802) -> (w3801:dbl[])
    n2890 = Bundle By Name(cluster=w3764, "Y"=w3763) -> (w3762:waveform(dbl))
    n2891 = Select(t=w3984, s=w3986, f=w3985) -> (s? t:f=w3983:dbl)
    n2892 = feedback-in #11(w3983) -> ()
    n2893 = Array Size(array=w3972) -> (size(s)=w3969:i32)
    n2894 = Array Size(array=w3698) -> (size(s)=w3971:i32)
    n2895 = local read "MCL Scanning"() -> (w3981:bool)
    n2896 = local read "APD Integration Time (s)"() -> (w3883:dbl)
    n2897 = Bundle(w3762, w3759) -> (w3758:cluster{waveform(dbl), waveform(dbl)})  [unwired: 1 out]
    n2898 = Build Array (concatenate)(w3876, w4007) -> (w3878:waveform(dbl)[])
    "All Signals" <- w3878
    n2899 = Split 1D Array(array=w3801, index=w3800) -> (first subarray=w3794:dbl[])  [unwired: 1 out]
    n2900 = feedback-in #14(w3794) -> ()
    n2901 = Multiply(x=w3971, y="APD Ave N") -> (x*y=w3970:dbl)
    n2902 = Greater?(x=w3969, y=w3970) -> (0:w3973:bool)
    n2903 = Not(x=w3986) -> (.not. x?=w3980:bool)
    n2904 = Cluster To Array(cluster=w3758) -> (array=w3734:waveform(dbl)[])
    "Trap Positions" <- w3734
    n2905 = To Double Precision Float(number=w3699) -> (double precision float=w3857:dbl[])
    n2906 = call-poly <vilib>:"Mean.vi"("X"=w3794) -> ("mean"=w3793:dbl)  [unwired: 1 out]
    "Mean T1 Position (nm)" <- w3793
    n2907 = Subtract(x=w3794, y=w3793) -> (x-y=w3799:dbl[])
    n2908 = Square(x=w3799) -> (x^2=w3798:dbl[])
    n2909 = And(x=w3980, y=w3981) -> (x .and. y?=w3982:bool)
    n2910 = call-poly <vilib>:"Mean.vi"("X"=w3798) -> ("mean"=w3797:dbl)  [unwired: 1 out]
    n2911 = case shown="True" w3973 {
      tunnel: w3972 -> [w4384 w4386]
      tunnel: [w4384 w4390] -> w3700
      tunnel: w3970 -> [_ w4388]
      tunnel: w3969 -> [_ w4391]
      tunnel: w3874 -> [w4383 w4385]
      tunnel: [w4383 w4387] -> w3701
      frame False {
      }
      frame True {
        n2912 = Subtract(x=w4391, y=w4388) -> (x-y=w4389:dbl)
        n2913 = Array Subset(array=w4386, index=w4389, length=w4388) -> (w4390:u32[])
        n2914 = Array Subset(array=w4385, index=w4389, length=w4388) -> (w4387:u32[])
      }
    }
    n2915 = feedback-in #12(w3700) -> ()
    n2916 = feedback-in #13(w3701) -> ()
    n2917 = Square Root(x=w3797) -> (sqrt(x)=w3796:dbl)
    n2918 = Or(x=w3982, y=w3978) -> (x .or. y?=w3979:bool)
    n2919 = Equal?(x="Tab Control 6", y=T41."High Res Display") -> (x = y?=w3914:bool)
    n2920 = Multiply(x="APD Disp. Scale", y=w3876) -> (x*y=w3885:waveform(dbl)[])
    n2921 = Multiply(x=10.0, y=w3796) -> (x*y=→"Trap 1 Position RMS (A)":dbl)
    n2922 = Multiply(x="APD Disp. Downsample", y=w3883) -> (x*y=w3881:dbl)
    n2923 = Divide(x=w3885, y=w3881) -> (x/y=w3855:waveform(dbl)[])
    n2924 = case "For displaying the high resolution display (no downsampling)" shown="True" w3914 {
      tunnel: w3880 -> [_ w4282]
      frame False {
      }
      frame True {
        n2925 = Index Array(array=w4282, index="High Res. Display") -> (element=w4283:waveform(dbl))
        n2926 = call <vilib>:"Std Deviation and Variance.vi"("X"=w4283) -> ("mean"=w4290:dbl, "standard deviation"=w4295:dbl)  [unwired: 1 in, 1 out]
        "Mean Intensity" <- w4290
        "Sigma" <- w4295
        n2927 = Subtract(x=w4283, y=w4290) -> (x-y=w4289:waveform(dbl))
        n2928 = Select(t=w4289, s="Subtract mean", f=w4283) -> (s? t:f=→"1 Channel":waveform(dbl))
        n2929 = Divide(x=w4295, y=w4290) -> (x/y=→"Sigma/Mean":dbl)
        n2930 = feedback #15(1) -> (w4284:i32)
        n2931 = Greater Or Equal?(x=w4284, y="Slow mean N ave.") -> (x >= y?=w4297:bool)
        n2932 = Increment(x=w4284) -> (x+1=w4299:i32)
        n2933 = Select(t=1, s=w4297, f=w4299) -> (s? t:f=w4286:i32)
        n2934 = feedback-in #15(w4286) -> ()
        n2935 = feedback #16() -> (w4287:waveform(dbl))  [unwired: 1 out]
        n2936 = case shown="Default" w4284 {
          tunnel: [w4302 w4305] -> w4288
          tunnel: w4287 -> [w4304 _]
          tunnel: w4283 -> [w4303 w4305]
          frame Default {
            n2937 = call-poly <vilib>:"Append Waveforms.vi"("waveform B"=w4303, "waveform A"=w4304) -> ("waveform out"=w4302:waveform(dbl))  [unwired: 1 in, 8 out]
          }
          frame 1 {
          }
        }
        n2938 = feedback-in #16(w4288) -> ()
        n2939 = case shown="True" w4297 {
          tunnel: w4288 -> [_ w4301]
          frame False {
          }
          frame True {
            n2940 = call-poly <vilib>:"Mean.vi"("X"=w4301) -> ("mean"=→"Slow mean":dbl)  [unwired: 1 out]
          }
        }
      }
    }
    n2941 = Index Array(array=w3855, index=0) -> (element=w3864:waveform(dbl))
    n2942 = Index Array(array=w3855, index=1) -> (element=w3862:waveform(dbl))
    n2943 = case "For computing FFTs for display" shown="True" "Compute FFT" {
      tunnel: w3880 -> [_ w4996]
      frame False {
      }
      frame True {
        n2944 = Build Array("FFT 1 Choice 1", "FFT 1 Choice 2", "FFT 2 Choice 1", "FFT 2 Choice 2") -> (w4989:u16[])
        n2945 = Array Size(array=w4996) -> (size(s)=w4995:i32)
        n2946 = feedback-in #17(w4989) -> ()
        n2947 = feedback #17(u16[] [100, 100, 100, 100]) -> (w4990:u16[])
        n2948 = feedback-in #18("# Spectra to Ave.") -> ()
        n2949 = feedback #18("# Spectra to Ave.") -> (w4987:dbl)
        n2950 = Not Equal?(x="# Spectra to Ave.", y=w4987) -> (x != y?=w4986:bool)
        n2951 = Not Equal?(x=w4989, y=w4990) -> (x != y?=w4988:bool)
        n2952 = feedback #19(1.0) -> (w4973:dbl)
        n2953 = Compound Arithmetic op=OR("Reset FFT", w4988, w4986) -> (w4971:bool)
        n2954 = Select(t=1.0, s=w4971, f=w4973) -> (s? t:f=w4975:dbl)
        n2955 = Greater?(x=w4975, y="# Spectra to Ave.") -> (0:w4994:bool)
        n2956 = Increment(x=w4975) -> (x+1=w4974:dbl)
        n2957 = feedback-in #19(w4974) -> ()
        n2958 = local read "DMA Update Period (s)"() -> (w4969:dbl)
        n2959 = Multiply(x="# Spectra to Ave.", y=w4969) -> (x*y=→"Ave. Time (s)":dbl)
        n2960 = Build Array(cluster{"f0":dbl, "df":dbl, "magnitude":dbl[]} {"f0"=0.0, "df"=0.0, "magnitude"=[]} ("PSD")) -> (w4978:cluster{"f0":dbl, "df":dbl, "magnitude":dbl[]}[])
        n2961 = Build Array(w4978, w4978, w4978, w4978) -> (w4980:T52)
        n2962 = feedback #20(w4980) -> (w4985:T52)
        n2963 = for {
          N: 4 -> [_]
          tunnel: w4989 -> [w5018] mode=indexing
          tunnel: w4996 -> [w5019]
          tunnel: w4995 -> [w5021]
          tunnel: w4971 -> [w5014]
          tunnel: w4994 -> [w5013]
          tunnel: "# Spectra to Ave." -> [w5012]
          tunnel: [w5011] -> w4984 mode=indexing
          tunnel: w4985 -> [w5016] mode=indexing
          tunnel: [w5015] -> w4972 mode=indexing
          tunnel: w4975 -> [w5010]
          n2964 = Less?(x=w5018, y=w5021) -> (x < y?=w5020:bool)
          n2965 = Index Array(array=w5019, index=w5018) -> (element=w5017:waveform(dbl))
          n2966 = case shown="True" w5020 {
            tunnel: w5017 -> [_ w5038]
            tunnel: w5016 -> [w5023 w5036]
            tunnel: [w5023 w5024] -> w5015
            tunnel: w5014 -> [_ w5035]
            tunnel: w5013 -> [_ w5028]
            tunnel: w5012 -> [_ w5027]
            tunnel: [cluster{"f0":dbl, "df":dbl, "magnitude":dbl[]} {"f0"=0.0, "df"=0.0, "magnitude"=[]} ("PSD") w5029] -> w5011
            tunnel: w5010 -> [_ w5026]
            frame False {
            }
            frame True {
              n2967 = call <vilib>:"Std Deviation and Variance.vi"("X"=w5038) -> ("mean"=w5039:dbl)  [unwired: 1 in, 2 out]
              n2968 = Subtract(x=w5038, y=w5039) -> (x-y=w5037:waveform(dbl))
              n2969 = xnode "Spectral Measurements"("Signals"=w5037) -> ("PSD"=w5031:cluster{"f0":dbl, "df":dbl, "magnitude":dbl[]})  [unwired: 1 in, 1 out]
              n2970 = case shown="False" w5035 {
                tunnel: w5036 -> [w5048 _]
                tunnel: [w5044 w5053] -> w5024
                tunnel: w5031 -> [w5047 w5054]
                tunnel: w5028 -> [w5046 _]
                frame False {
                  n2971 = Build Array (concatenate)(w5048, w5047) -> (w5045:cluster{"f0":dbl, "df":dbl, "magnitude":dbl[]}[])
                  n2972 = case shown="True" w5046 {
                    tunnel: w5045 -> [w5049 w5052]
                    tunnel: [w5049 w5050] -> w5044
                    frame False {
                    }
                    frame True {
                      n2973 = Delete From Array(array=w5052, index=0) -> (array with subset deleted=w5050:cluster{"f0":dbl, "df":dbl, "magnitude":dbl[]}[])  [unwired: 1 in, 1 out]
                    }
                  }
                }
                frame True {
                  n2974 = Build Array(w5054) -> (w5053:cluster{"f0":dbl, "df":dbl, "magnitude":dbl[]}[])
                }
              }
              n2975 = for {
                tunnel: w5024 -> [w5043] mode=indexing
                tunnel: [w5042] -> w5034 mode=indexing
                workers-P: _ -> [_]
                n2976 = Unbundle By Name(w5043) -> ("magnitude"=w5042:dbl[])
              }
              n2977 = Transpose 2D Array(2D array=w5034) -> (transposed array=w5033:dbl[][])
              n2978 = for {
                tunnel: w5033 -> [w5041] mode=indexing
                tunnel: [w5040] -> w5032 mode=indexing
                workers-P: _ -> [_]
                n2979 = Add Array Elements(numeric array=w5041) -> (sum=w5040:dbl)
              }
              n2980 = Select(t=w5027, s=w5028, f=w5026) -> (s? t:f=w5025:dbl)
              n2981 = Divide(x=w5032, y=w5025) -> (x/y=w5030:dbl[])
              n2982 = Bundle By Name(cluster=w5031, "magnitude"=w5030) -> (w5029:cluster{"f0":dbl, "df":dbl, "magnitude":dbl[]})
            }
          }
        }
        n2983 = case shown="True" w4971 {
          tunnel: w4972 -> [w5003 w5009]
          tunnel: [w5003 w5004] -> w4970
          frame False {
          }
          frame True {
            n2984 = Array Subset(array=w5009, index (row)=0 ("index"), length (row)=4 ("length"), index (col)=0 ("index"), length (col)=1 ("length")) -> (w5004:T52)
          }
        }
        n2985 = feedback-in #20(w4970) -> ()
        n2986 = Split 1D Array(array=w4984, index=2) -> (first subarray=→"FFT 1":cluster{"f0":dbl, "df":dbl, "magnitude":dbl[]}[], second subarray=→"FFT 2":cluster{"f0":dbl, "df":dbl, "magnitude":dbl[]}[])
      }
    }
    n2987 = case "For plotting results of scanning MCL" shown="True" w3979 {
      tunnel: w3978 -> [_ w4424]
      tunnel: w3908 -> [_ w4520]
      tunnel: w3987 -> [_ _]
      tunnel: w3880 -> [_ w4494]
      tunnel: w3857 -> [_ w4425]
      tunnel: w3856 -> [_ w4398]
      frame False {
      }
      frame True {
        w4405 = u32 0 items=["Horizontal", "Vertical", "Central", "1st Diagonal", "2nd Diagonal"] ("Type of Symmetry")
        w4433 = u32 0 items=["Horizontal", "Vertical", "Central", "1st Diagonal", "2nd Diagonal"] ("Type of Symmetry")
        w4436 = u32 0 items=["Horizontal", "Vertical", "Central", "1st Diagonal", "2nd Diagonal"] ("Type of Symmetry")
        w4465 = u32 0 items=["Horizontal", "Vertical", "Central", "1st Diagonal", "2nd Diagonal"] ("Type of Symmetry")
        n2988 = Index Array(array=w4494, index=10) -> (element=w4500:waveform(dbl))
        n2989 = Index Array(array=w4494, index=11) -> (element=w4497:waveform(dbl))
        n2990 = local read "Cycles/step (MCL)"() -> (w4450:u64)
        n2991 = Index Array(array=w4494, index="Channel") -> (element=w4496:waveform(dbl))
        n2992 = Unbundle(w4398) -> ("New Image"=w4397:T2, "New Image"=w4396:T2, "New Image"=w4395:T2, "New Image"=w4394:T2)
        n2993 = Unbundle By Name(w4500) -> ("Y"=w4452:dbl[])
        n2994 = Unbundle By Name(w4497) -> ("Y"=w4454:dbl[])
        n2995 = Unbundle By Name(w4496) -> ("Y"=w4459:dbl[])
        n2996 = call "downsample 1D array - double.vi"("Ave N"=w4450, "Array In"=w4452) -> ("Array Out"=w4451:dbl[])  [unwired: 1 out]
        n2997 = call "downsample 1D array - double.vi"("Ave N"=w4450, "Array In"=w4454) -> ("Array Out"=w4453:dbl[])  [unwired: 1 out]
        n2998 = call "downsample 1D array - double.vi"("Ave N"=w4450, "Array In"=w4459) -> ("Array Out"=w4458:dbl[])  [unwired: 1 out]
        n2999 = feedback #21(w4520) -> (w4521:dbl[])
        n3000 = Build Array (concatenate)(w4521, w4520) -> (w4502:dbl[])
        n3001 = feedback #22(w4425) -> (w4427:dbl[])
        n3002 = Build Array (concatenate)(w4427, w4425) -> (w4426:dbl[])
        n3003 = local read "Scan steps (MCL)"() -> (w4407:u64)
        n3004 = Select(t=w4520, s=w4424, f=w4502) -> (s? t:f=w4506:dbl[])
        n3005 = feedback-in #21(w4506) -> ()
        n3006 = Select(t=w4425, s=w4424, f=w4426) -> (s? t:f=w4408:dbl[])
        n3007 = feedback-in #22(w4408) -> ()
        n3008 = local read "Scan lines (y)"() -> (w4393:u64)
        n3009 = local read "N APD Samp/step"() -> (w4409:dbl)
        n3010 = feedback #23(w4451) -> (w4508:dbl[])
        n3011 = Build Array (concatenate)(w4508, w4451) -> (w4499:dbl[])
        n3012 = feedback #24(w4458) -> (w4518:dbl[])
        n3013 = Build Array (concatenate)(w4518, w4458) -> (w4517:dbl[])
        n3014 = feedback #25(w4453) -> (w4510:dbl[])
        n3015 = Build Array (concatenate)(w4510, w4453) -> (w4511:dbl[])
        n3016 = Select(t=w4451, s=w4424, f=w4499) -> (s? t:f=w4455:dbl[])
        n3017 = feedback-in #23(w4455) -> ()
        n3018 = Select(t=w4458, s=w4424, f=w4517) -> (s? t:f=w4457:dbl[])
        n3019 = feedback-in #24(w4457) -> ()
        n3020 = Select(t=w4453, s=w4424, f=w4511) -> (s? t:f=w4456:dbl[])
        n3021 = feedback-in #25(w4456) -> ()
        n3022 = Multiply(x=w4407, y=u64 2) -> (x*y=w4392:u64)
        n3023 = call "integrate 1D array interval - double.vi"("Ave N"=w4409, "Array In"=w4408) -> ("Array Out"=w4420:dbl[])  [unwired: 1 out]
        n3024 = call "integrate 1D array interval - double.vi"("Ave N"=w4409, "Array In"=w4506) -> ("Array Out"=w4505:dbl[])  [unwired: 1 out]
        n3025 = Array Size(array=w4420) -> (size(s)=w4421:i32)
        n3026 = Array Size(array=w4505) -> (size(s)=w4507:i32)
        n3027 = Multiply(x=w4393, y=w4392) -> (x*y=w4423:u64)
        n3028 = Multiply(x=w4393, y=w4392) -> (x*y=w4515:u64)
        n3029 = call-poly <vilib>:"Mean.vi"("X"=w4455) -> ("mean"=w4439:dbl)  [unwired: 1 out]
        n3030 = Subtract(x=w4423, y=w4421) -> (x-y=w4414:u64)
        n3031 = call-poly <vilib>:"Mean.vi"("X"=w4457) -> ("mean"=w4444:dbl)  [unwired: 1 out]
        n3032 = call-poly <vilib>:"Mean.vi"("X"=w4456) -> ("mean"=w4442:dbl)  [unwired: 1 out]
        n3033 = call-poly <vilib>:"Mean.vi"("X"=w4420) -> ("mean"=w4411:dbl)  [unwired: 1 out]
        n3034 = Subtract(x=w4515, y=w4507) -> (x-y=w4449:u64)
        n3035 = call-poly <vilib>:"Mean.vi"("X"=w4505) -> ("mean"=w4446:dbl)  [unwired: 1 out]
        n3036 = Initialize Array(1.0 ("element"), w4414) -> (w4410:dbl[])
        n3037 = Initialize Array(1.0 ("element"), w4449) -> (w4440:dbl[])
        n3038 = Multiply(x=w4410, y=w4411) -> (x*y=w4412:dbl[])
        n3039 = Multiply(x=w4440, y=w4442) -> (x*y=w4443:dbl[])
        n3040 = Multiply(x=w4440, y=w4444) -> (x*y=w4445:dbl[])
        n3041 = Multiply(x=w4440, y=w4439) -> (x*y=w4441:dbl[])
        n3042 = Multiply(x=w4440, y=w4446) -> (x*y=w4447:dbl[])
        n3043 = Build Array (concatenate)(w4455, w4441) -> (w4509:dbl[])
        n3044 = Build Array (concatenate)(w4457, w4445) -> (w4513:dbl[])
        n3045 = Build Array (concatenate)(w4456, w4443) -> (w4512:dbl[])
        n3046 = Build Array (concatenate)(w4420, w4412) -> (w4422:dbl[])
        n3047 = Build Array (concatenate)(w4505, w4447) -> (w4514:dbl[])
        n3048 = Reshape Array(w4509, w4393, w4392) -> (w4475:dbl[][])
        n3049 = Reshape Array(w4422, w4393, w4392) -> (w4418:dbl[][])
        n3050 = Reshape Array(w4513, w4393, w4392) -> (w4467:dbl[][])
        n3051 = Reshape Array(w4512, w4393, w4392) -> (w4482:dbl[][])
        n3052 = Reshape Array(w4514, w4393, w4392) -> (w4492:dbl[][])
        n3053 = Array Subset(array=w4482, index (col)=0 ("index"), length (col)=w4407) -> (w4487:dbl[][])  [unwired: 2 in]
        n3054 = Array Subset(array=w4482, index (col)=w4407) -> (w4485:dbl[][])  [unwired: 3 in]
        n3055 = Array Subset(array=w4467, index (col)=0 ("index"), length (col)=w4407) -> (w4473:dbl[][])  [unwired: 2 in]
        n3056 = Array Subset(array=w4467, index (col)=w4407) -> (w4471:dbl[][])  [unwired: 3 in]
        n3057 = Array Subset(array=w4418, index (col)=0 ("index"), length (col)=w4407) -> (w4417:dbl[][])  [unwired: 2 in]
        n3058 = Array Subset(array=w4418, index (col)=w4407) -> (w4415:dbl[][])  [unwired: 3 in]
        n3059 = Array Subset(array=w4492, index (col)=0 ("index"), length (col)=w4407) -> (w4491:dbl[][])  [unwired: 2 in]
        n3060 = Array Subset(array=w4492, index (col)=w4407) -> (w4489:dbl[][])  [unwired: 3 in]
        n3061 = Array Subset(array=w4475, index (col)=0 ("index"), length (col)=w4407) -> (w4480:dbl[][])  [unwired: 2 in]
        n3062 = Array Subset(array=w4475, index (col)=w4407) -> (w4478:dbl[][])  [unwired: 3 in]
        n3063 = for {
          tunnel: w4487 -> [w4529] mode=indexing
          tunnel: [w4528] -> w4486 mode=indexing
          workers-P: _ -> [_]
          n3064 = Reverse 1D Array(array=w4529) -> (reversed array=w4528:dbl[])
        }
        n3065 = for {
          tunnel: w4473 -> [w4525] mode=indexing
          tunnel: [w4524] -> w4472 mode=indexing
          workers-P: _ -> [_]
          n3066 = Reverse 1D Array(array=w4525) -> (reversed array=w4524:dbl[])
        }
        n3067 = for {
          tunnel: w4417 -> [w4523] mode=indexing
          tunnel: [w4522] -> w4416 mode=indexing
          workers-P: _ -> [_]
          n3068 = Reverse 1D Array(array=w4523) -> (reversed array=w4522:dbl[])
        }
        n3069 = for {
          tunnel: w4491 -> [w4531] mode=indexing
          tunnel: [w4530] -> w4490 mode=indexing
          workers-P: _ -> [_]
          n3070 = Reverse 1D Array(array=w4531) -> (reversed array=w4530:dbl[])
        }
        n3071 = for {
          tunnel: w4480 -> [w4527] mode=indexing
          tunnel: [w4526] -> w4479 mode=indexing
          workers-P: _ -> [_]
          n3072 = Reverse 1D Array(array=w4527) -> (reversed array=w4526:dbl[])
        }
        n3073 = Index Array(array=w4492, index (row)=0) -> (element=→"Waveform Graph":dbl[])  [unwired: 1 in]
        n3074 = Add(x=w4486, y=w4485) -> (x+y=w4484:dbl[][])
        n3075 = Add(x=w4472, y=w4471) -> (x+y=w4470:dbl[][])
        n3076 = Add(x=w4416, y=w4415) -> (x+y=w4400:dbl[][])
        n3077 = Add(x=w4490, y=w4489) -> (x+y=w4464:dbl[][])
        n3078 = Add(x=w4479, y=w4478) -> (x+y=w4477:dbl[][])
        n3079 = Divide(x=w4470, y=2) -> (x/y=w4468:dbl[][])
        n3080 = Divide(x=w4484, y=2) -> (x/y=w4429:dbl[][])
        n3081 = Divide(x=w4477, y=2) -> (x/y=w4431:dbl[][])
        n3082 = To Single Precision Float(number=w4464) -> (single precision float=w4463:sgl[][])
        n3083 = Transpose 2D Array(2D array=w4468) -> (transposed array=→"Data map":dbl[][])
        n3084 = To Single Precision Float(number=w4400) -> (single precision float=w4404:sgl[][])
        n3085 = To Single Precision Float(number=w4429) -> (single precision float=w4435:sgl[][])
        n3086 = To Single Precision Float(number=w4431) -> (single precision float=w4432:sgl[][])
        n3087 = call "IMAQ ArrayToImage"("Image Pixels (Float)"=w4463, "Image"=w4397) -> ("Image Out"=w4466:T2)  [unwired: 8 in, 1 out]
        n3088 = call "IMAQ ArrayToImage"("Image Pixels (Float)"=w4404, "Image"=w4396) -> ("Image Out"=w4406:T2)  [unwired: 8 in, 1 out]
        n3089 = call "IMAQ ArrayToImage"("Image Pixels (Float)"=w4435, "Image"=w4395) -> ("Image Out"=w4437:T2)  [unwired: 8 in, 1 out]
        n3090 = call "IMAQ ArrayToImage"("Image Pixels (Float)"=w4432, "Image"=w4394) -> ("Image Out"=w4434:T2)  [unwired: 8 in, 1 out]
        n3091 = call "IMAQ Symmetry"("Type of Symmetry"=w4465, "Image Src"=w4466) -> ("Image Dst Out"=w4461:T2)  [unwired: 3 in, 1 out]
        n3092 = call "IMAQ Symmetry"("Type of Symmetry"=w4405, "Image Src"=w4406) -> ("Image Dst Out"=w4402:T2)  [unwired: 3 in, 1 out]
        n3093 = call "IMAQ Symmetry"("Type of Symmetry"=w4436, "Image Src"=w4437) -> ("Image Dst Out"=→"Detection Laser X":T2)  [unwired: 3 in, 1 out]
        n3094 = call "IMAQ Symmetry"("Type of Symmetry"=w4433, "Image Src"=w4434) -> ("Image Dst Out"=→"Detection Laser Y":T2)  [unwired: 3 in, 1 out]
        n3095 = call "IMAQ Set Simple Calibration"("Calibration Axis Info"=T42 {"Origin Pixel"={"X"=0.0, "Y"=0.0}, "Angle Relative to Horizontal (deg)"=0.0, "Axis Reference"=0}, "Grid Descriptor"=T43 {"X Step"=0.3, "Y Step"=0.3, "Unit"=enum."Undefined"}, "Image"=w4461) -> ("Calibrated Image"=→"APD 1":T2)  [unwired: 7 in, 1 out]
        n3096 = call "IMAQ Set Simple Calibration"("Calibration Axis Info"=T42 {"Origin Pixel"={"X"=0.0, "Y"=0.0}, "Angle Relative to Horizontal (deg)"=0.0, "Axis Reference"=0}, "Grid Descriptor"=T43 {"X Step"=0.3, "Y Step"=0.3, "Unit"=enum."Undefined"}, "Image"=w4402) -> ("Calibrated Image"=→"APD 2":T2)  [unwired: 7 in, 1 out]
      }
    }
    n3097 = Subtract(x=w3862, y="APD 2 Offset") -> (x-y=w3859:waveform(dbl))
    n3098 = Subtract(x=w3864, y="APD 1 Offset") -> (x-y=w3860:waveform(dbl))
    n3099 = Index Array(array=w3878, index=3) -> (element=w3932:waveform(dbl))
    n3100 = Index Array(array=w3878, index=6) -> (element=w3929:waveform(dbl))
    n3101 = Build Array(w3860, w3859) -> (→"APD Chart":waveform(dbl)[])
    n3102 = Array Size(array=w3700) -> (size(s)=w3968:i32)
    n3103 = call <vilib>:"Std Deviation and Variance.vi"("X"=w3701) -> ("standard deviation"=w3871:dbl)  [unwired: 1 in, 2 out]
    n3104 = Add Array Elements(numeric array=w3701) -> (sum=w3873:u32)
    n3105 = Add Array Elements(numeric array=w3700) -> (sum=w3977:u32)
    n3106 = call <vilib>:"Std Deviation and Variance.vi"("X"=w3700) -> ("standard deviation"=w3923:dbl)  [unwired: 1 in, 2 out]
    n3107 = Divide(x="T1 offset_x (mV)", y=1000.0) -> (x/y=w3933:dbl)
    n3108 = Divide(x=w3871, y=w3870) -> (x/y=w3867:dbl)
    "Rate sigma (Hz) 2" <- w3867
    n3109 = Multiply(x=w3870, y=w3968) -> (x*y=w3872:dbl)
    "Int. Time (s)" <- w3872
    n3110 = Divide(x=w3873, y=w3872) -> (x/y=w3868:dbl)
    "APD 2 Rate (Hz)" <- w3868
    n3111 = Divide(x=w3977, y=w3872) -> (x/y=w3921:dbl)
    "APD 1 Rate (Hz)" <- w3921
    n3112 = Divide(x=w3923, y=w3870) -> (x/y=w3922:dbl)
    "Rate sigma (Hz)" <- w3922
    n3113 = Divide(x=w3867, y=w3868) -> (x/y=→"Sigma/Mean 2":dbl)
    n3114 = Divide(x=w3922, y=w3921) -> (x/y=→"s/Mean":dbl)
    n3115 = feedback-in #26("Calibration") -> ()
    n3116 = feedback #26(u16 1 ("Calibration")) -> (w3951:u16)
    n3117 = Divide(x="T2 offset_x (mV)", y=1000.0) -> (x/y=w3931:dbl)
    n3118 = case shown="0, Default" "Calibration" {
      tunnel: "T1 a_x (nm/V)" -> [_ w4360 w4381]
      tunnel: "T1 k_x (pN/nm)" -> [_ _ w4371]
      tunnel: "T2 a_x (nm/V)" -> [_ w4359 w4379]
      tunnel: "T2 k_x (pN/nm)" -> [_ _ w4372]
      tunnel: w3932 -> [w4342 w4357 w4377]
      tunnel: w3929 -> [w4341 w4355 w4375]
      tunnel: [w4342 w4354 w4374] -> w3960
      tunnel: [w4341 w4353 w4373] -> w3959
      tunnel: ["T1 X (V)" ("Label.Text") "T1 X (nm)" ("Label.Text") "T1 X (pN)" ("Label.Text")] -> w3948
      tunnel: ["T2 X (V)" ("Label.Text") "T2 X (nm)" ("Label.Text") "T2 X (pN)" ("Label.Text")] -> w3947
      tunnel: ["Position (V)" ("Label.Text") "Position (nm)" ("Label.Text") "Force (pN)" ("Label.Text")] -> w3949
      tunnel: w3931 -> [_ w4345 w4364]
      tunnel: w3933 -> [_ w4348 w4366]
      tunnel: ["Mean (V)" ("Label.Text") "Mean (nm)" ("Label.Text") "Mean (pN)" ("Label.Text")] -> w3944
      tunnel: ["Difference (V)" ("Label.Text") "Difference (nm)" ("Label.Text") "Difference (pN)" ("Label.Text")] -> w3886
      frame 0, Default {
      }
      frame 1 {
        n3119 = Unbundle By Name(w4357) -> ("Y"=w4361:dbl[])
        n3120 = Unbundle By Name(w4355) -> ("Y"=w4346:dbl[])
        n3121 = Subtract(x=w4361, y=w4348) -> (x-y=w4349:dbl[])
        n3122 = Subtract(x=w4346, y=w4345) -> (x-y=w4347:dbl[])
        n3123 = Multiply(x=w4347, y=w4359) -> (x*y=w4356:dbl[])
        n3124 = Multiply(x=w4360, y=w4349) -> (x*y=w4358:dbl[])
        n3125 = Bundle By Name(cluster=w4355, "Y"=w4356) -> (w4353:waveform(dbl))
        n3126 = Bundle By Name(cluster=w4357, "Y"=w4358) -> (w4354:waveform(dbl))
      }
      frame 2 {
        n3127 = Unbundle By Name(w4377) -> ("Y"=w4382:dbl[])
        n3128 = Unbundle By Name(w4375) -> ("Y"=w4380:dbl[])
        n3129 = Subtract(x=w4380, y=w4364) -> (x-y=w4365:dbl[])
        n3130 = Subtract(x=w4382, y=w4366) -> (x-y=w4367:dbl[])
        n3131 = Compound Arithmetic op=MULTIPLY(w4365, w4379, w4372) -> (w4376:dbl[])
        n3132 = Compound Arithmetic op=MULTIPLY(w4371, w4381, w4367) -> (w4378:dbl[])
        n3133 = Bundle By Name(cluster=w4375, "Y"=w4376) -> (w4373:waveform(dbl))
        n3134 = Bundle By Name(cluster=w4377, "Y"=w4378) -> (w4374:waveform(dbl))
      }
    }
    n3135 = Not Equal?(x=w3951, y="Calibration") -> (x != y?=w3912:bool)
    n3136 = case shown="True" w3912 {
      tunnel: w3949 -> [_ w4335]
      tunnel: w3948 -> [_ w4334]
      tunnel: w3947 -> [_ w4333]
      tunnel: w3944 -> [_ w4332]
      tunnel: w3886 -> [_ w4331]
      frame False {
      }
      frame True {
        n3137 = property on="Force" class="WFChart (strict)"("YScale.NameLbl.Text"=w4335) -> ()  [unwired: 2 in, 2 out]
        n3138 = property on="T2 X" class="DigNum (strict)"("Caption.Text"=w4333) -> ()  [unwired: 2 in, 2 out]
        n3139 = property on="T1 X" class="DigNum (strict)"("Caption.Text"=w4334) -> ()  [unwired: 2 in, 2 out]
        n3140 = property on="Mean" class="DigNum (strict)"("Caption.Text"=w4332) -> ()  [unwired: 2 in, 2 out]
        n3141 = property on="Difference" class="DigNum (strict)"("Caption.Text"=w4331) -> ()  [unwired: 2 in, 2 out]